vi "Minhee Analysis_new.vi"(4 "Polarity":T2 items=["Inward", "Outward"], 5 "Data type":T1 items=["AXON", "HEKA"], 6 "Sweep length":dbl=51662.0, 7 "Path of File":path=path "C:/Users/KimYG/Desktop/test4.abf") -> ()   [LabVIEW 2017]
uses:
  <vilib>/Analysis/NI_AALBase.lvlib
  <vilib>/addons/_Advanced Signal Processing/NI_AdvSigProcWA.lvlib
  <vilib>/Utility/file.llb/Write Delimited Spreadsheet (DBL).vi
  <vilib>/Utility/miscctls.llb/LVRowAndColumnTypeDef.ctl
  <vilib>/Analysis/3filter.llb/Savitzky-Golay Filter (DBL).vi
  <vilib>/addons/Wavelet Analysis/application.llb/WA Multiscale Peak Detection (Array).vi
  Event Detection cluster.ctl
  <vilib>/Analysis/baseanly.llb/Mean (DBL).vi
  Minhee analysis parameter setting.ctl
  Polarity.ctl
  Data type_new.ctl
panel:
  out "Holding Current":dbl[](graph)
  out "Mean Frequency":string caption="String"
  out "Sweep duration":dbl
  in  "Clipboard":bool
  out "Number of event":i32[][](graph)
  out "Selected event":string caption="String"
  out "Pining point":string caption="String"
  out "Mean IEI":string caption="String"
  out "Mean Amplitude":string caption="String"
  out "Total event":string caption="String"
  in  "Pin here":bool
  in  "Raw trace":bool
  out "Distribution of amplitude 2":T3(graph) caption="Selected"
  out "Distribution of IEI 2":T3(graph) caption="Selected"
  out "Mean IEI":string caption="String"
  out "Mean Amplitude":string caption="String"
  out "CV":dbl[](graph)
  in  "Baseline selection":T4(ring)
  in  "Screening":bool
  out "dv/dt":cluster{"X (time)":dbl[], "dX/dt":dbl[]}[](graph)
  in  "Save":bool
  out "Distribution of amplitude":T3(graph) caption="Total"
  out "Distribution of IEI":T3(graph) caption="Total"
  in  "Event #":i16=4 min=0 max=15 step=1
  out "Event":cluster{dbl[], dbl[]}[](graph)
  in  "Delete":bool
  in  "Do it":bool
  in  "Parameter setting":T5={"Event Detection Parameter"={"Threshold"=-10.0, "width "=20}, "Smoothing Parameter"={"polynomial order"=3, "side points"=20}, "Screening threshold (dV/dt)"=-6000.0, "Screening threshold (amplitude)"=-10.0} {"Screening threshold (amplitude)" format="%#_13g"; "Event Detection Parameter"."Threshold" format="%#_13g"}
  in  "정지":bool
  in  "Sweep #":i32 min=0 max=49 step=1
  out "Detected Event":string[][](table)
  out "Original trace":cluster{"Ramp Pattern":dbl[], "X":dbl[]}[](graph)
  # "Event Table"
  # "Sweep Info."
  # "Data file configuration"
  # "Parameter setting"
  # "Action"
  # "Search parameter"
  # "Home"
  # "Pg Up"
  # "End"
  # "Pg Dn"
  # "Result - Total & Representative (200 events)"
  # "Minhee Analysis for sEPSC/sIPSC"
  # "Whole trace"
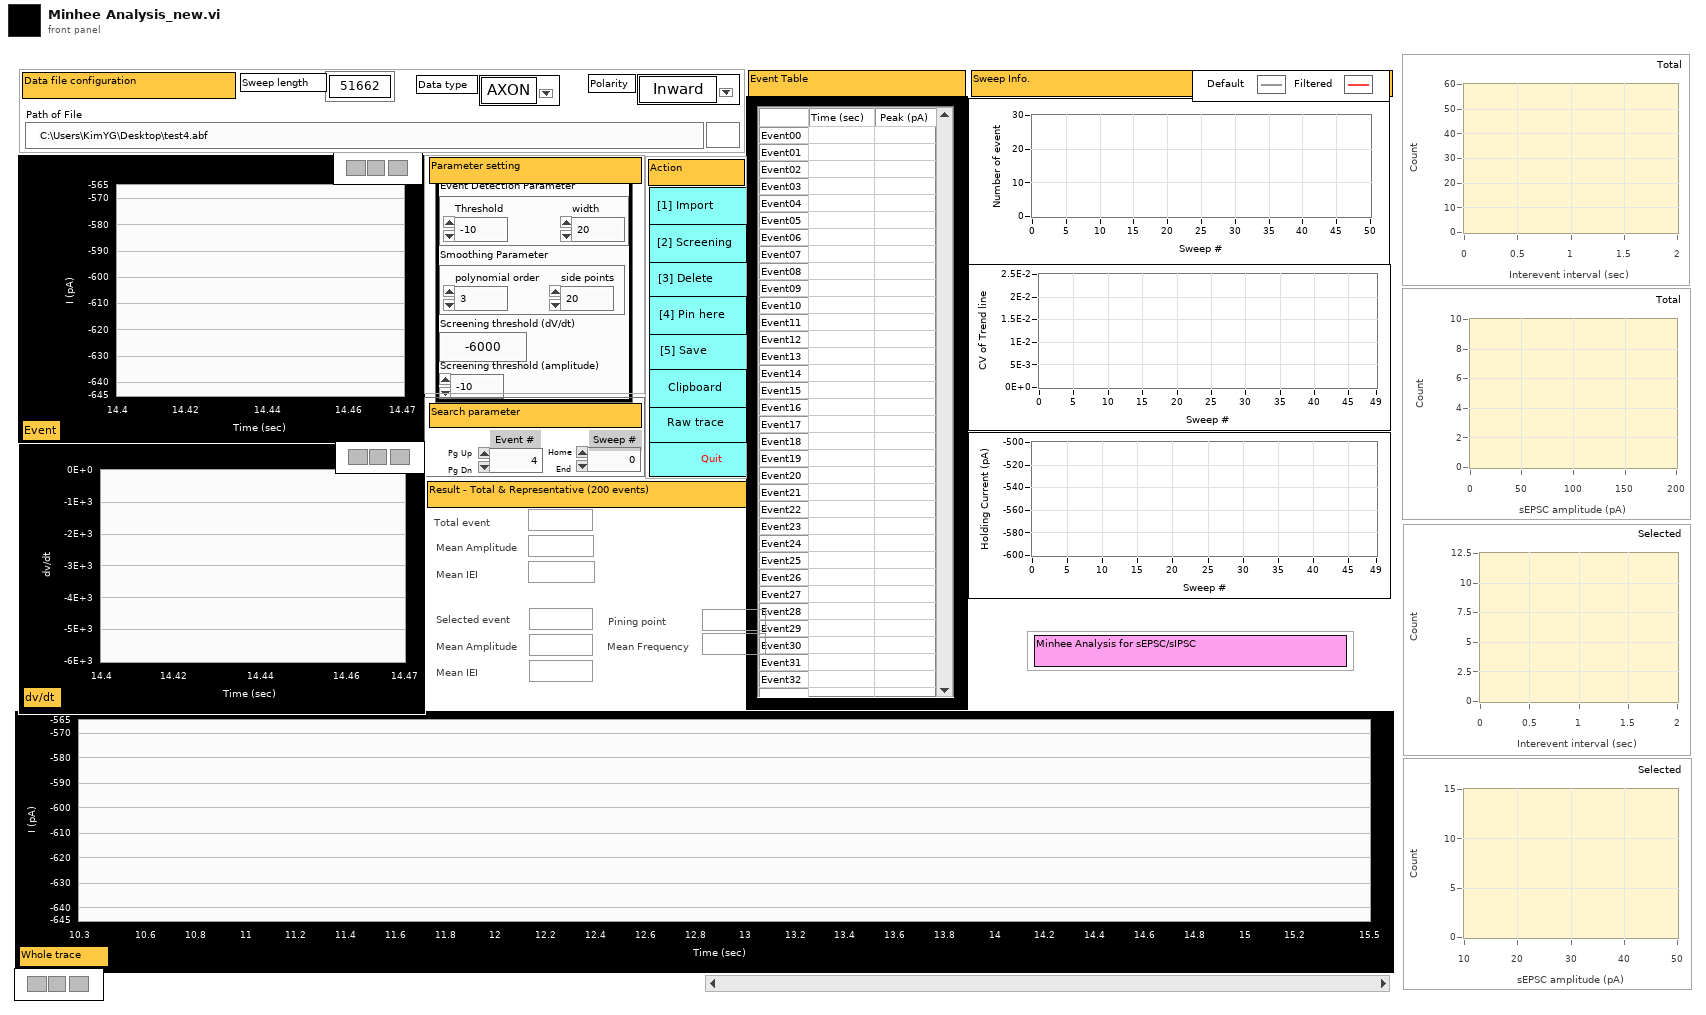
[diagram p1: front panel]
types:
  T1 = typedef "Data type_new.ctl" = u16
  T2 = typedef "Polarity.ctl" = u16
  T3 = cluster{"X Values":dbl[], "Histogram: h(x)":i32[]}
  T4 = enum16{"Adjusted baseline", "Trend line", "Previously used"}
  T5 = typedef "Minhee analysis parameter setting.ctl" = cluster{"Event Detection Parameter":cluster{"Threshold":dbl, "width ":i32}, "Smoothing Parameter":cluster{"polynomial order":i32, "side points":i32}, "Screening threshold (dV/dt)":dbl, "Screening threshold (amplitude)":dbl}
  T6 = typedef "Event Detection cluster.ctl" = cluster{"Event (1D)":cluster{"Event time":dbl[], "Event Peak":dbl[]}, "Trace (1D)":cluster{"Trace time":dbl[], "Trace":dbl[]}, "Trend (1D)":cluster{"Trend time":dbl[], "Trend":dbl[]}, "Baseline (1D)":cluster{"Baseline time":dbl[], "Baseline":dbl[]}}
  T7 = cluster{"Total":cluster{"Distribution of IEI":cluster{"X Values":dbl[], "Histogram: h(x)":i32[]}, "Distribution of amplitude":cluster{"X Values":dbl[], "Histogram: h(x)":i32[]}, "Total":cluster{"EVT #":string, "Amplitude":string, "IEI":string}, "Number of event":i32[]}, "Selected":cluster{"Distribution of IEI ":cluster{"X Values":dbl[], "Histogram: h(x)":i32[]}, "Distribution of amplitude":cluster{"X Values":dbl[], "Histogram: h(x)":i32[]}, "Selected":cluster{"EVT #":string, "Amplitude":string, "IEI":string, "Frequency":string}}}
  T8 = cluster{"X (time)":dbl[], "I (pA)":dbl[], "dX/dt":dbl[]}
  T9 = cluster{"Distribution of IEI ":cluster{"X Values":dbl[], "Histogram: h(x)":i32[]}, "Distribution of amplitude":cluster{"X Values":dbl[], "Histogram: h(x)":i32[]}, "Selected":cluster{"EVT #":string, "Amplitude":string, "IEI":string, "Frequency":string}}
  T10 = cluster{"detrend? (F)":bool, "threshold frequency":dbl}
  T11 = typedef "LVRowAndColumnTypeDef.ctl" = cluster{"Row":i32, "Column":i32}
  T12 = cluster{"File Path":path, "Cell ID":string, "File Name":string, "Total Length":i32, "Trial Length (ms)":dbl, "Sweep Number":dbl, "Sampling rate":dbl}
  T13 = cluster{"polynomial order":i32, "side points":i32}
  T14 = cluster{"Path of File":path, "Sweep length ":dbl, "Data type":T1}
  T15 = cluster{"Histogram Graph":cluster{"X Values":dbl[], "Histogram: h(x)":i32[]}, "Histogram Graph":cluster{"X Values":dbl[], "Histogram: h(x)":i32[]}, cluster{"EVT #":string, "Mean amplitude":string, "Mean IEI":string, "Mean frequency":string}}
  T16 = typedef "Baseline selection.ctl" = enum16{"Default", "Manual"}
  T17 = cluster{"Histogram Graph":cluster{"X Values":dbl[], "Histogram: h(x)":i32[]}, "Histogram Graph":cluster{"X Values":dbl[], "Histogram: h(x)":i32[]}, cluster{string, "standard deviation":string, "standard deviation":string}, i32[]}
  T18 = cluster{"EVT #":string, "Amplitude":string, "IEI":string}
  T19 = cluster{"EVT #":string, "Amplitude":string, "IEI":string, "Frequency":string}
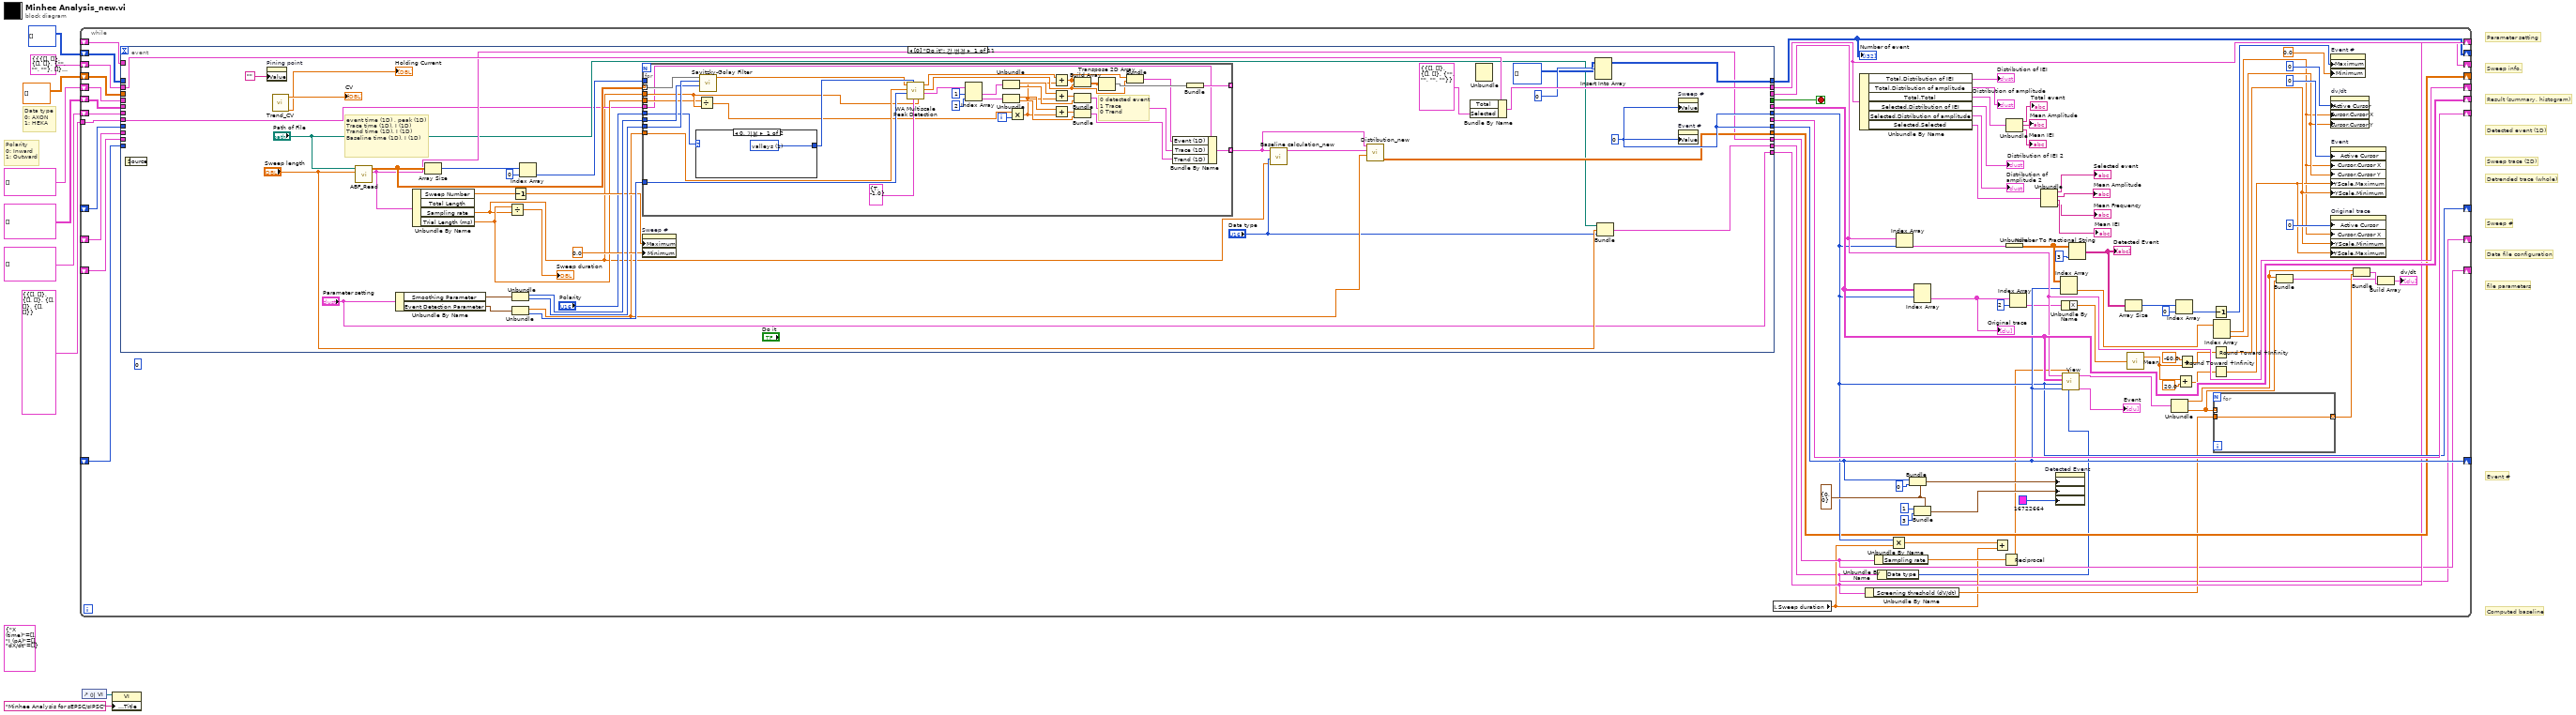
[diagram p0: block diagram]
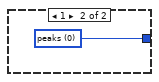
[diagram p2: hidden frame]
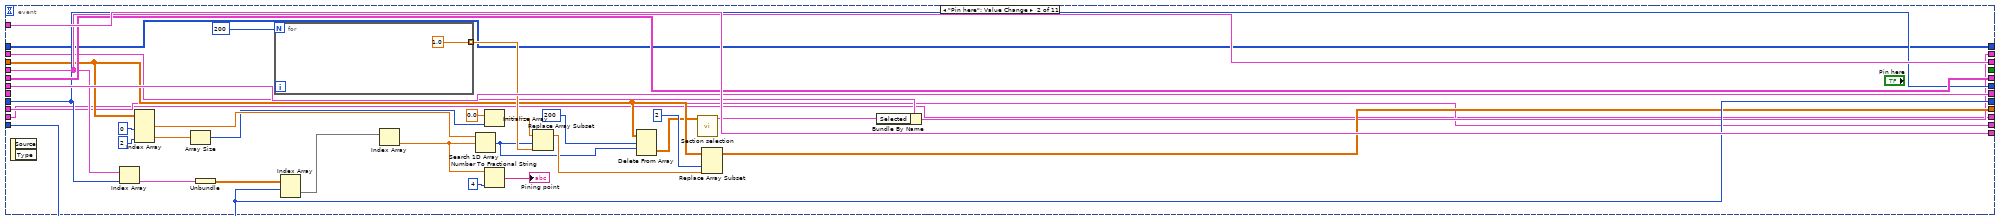
[diagram p3: hidden frame]
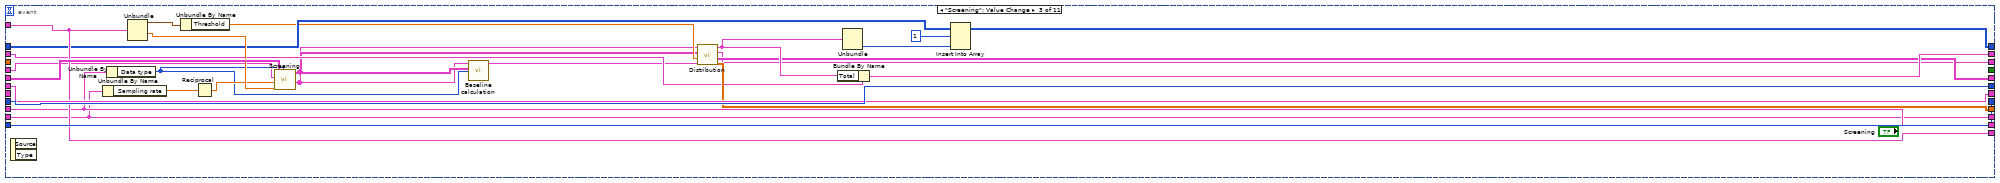
[diagram p4: hidden frame]
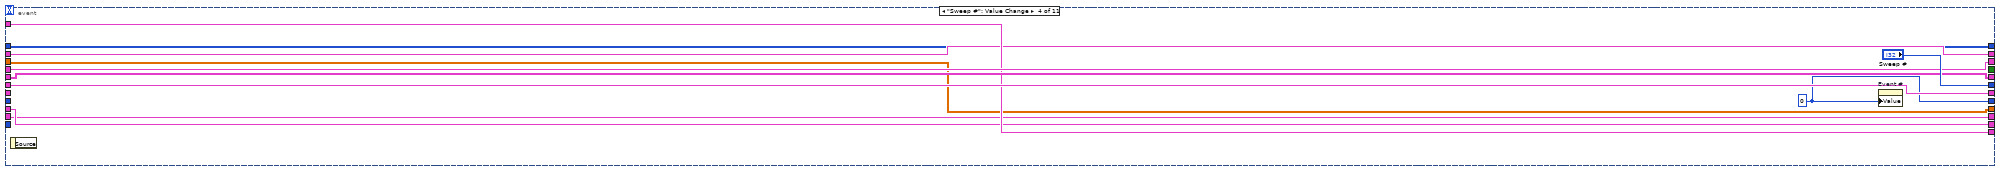
[diagram p5: hidden frame]
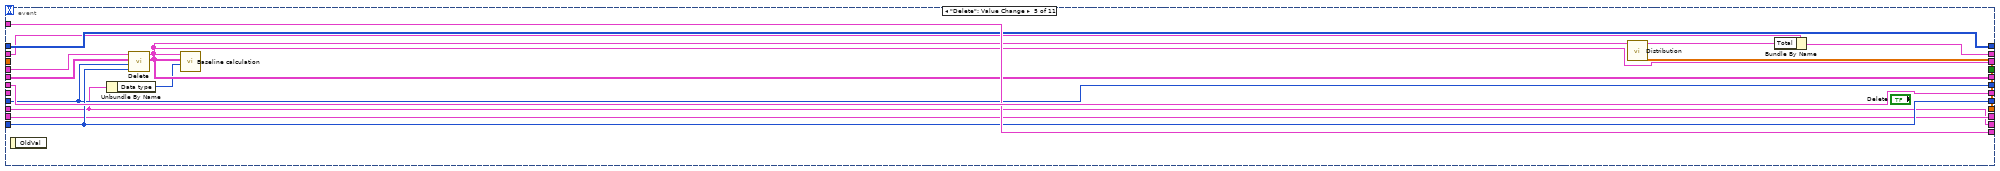
[diagram p6: hidden frame]
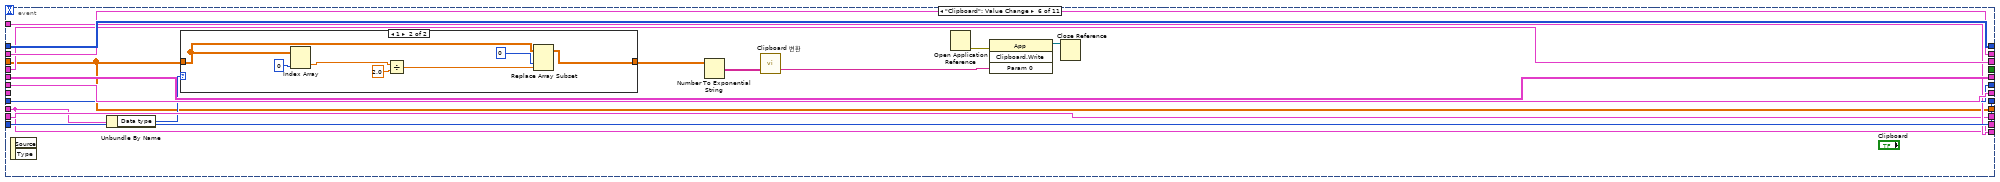
[diagram p7: hidden frame]
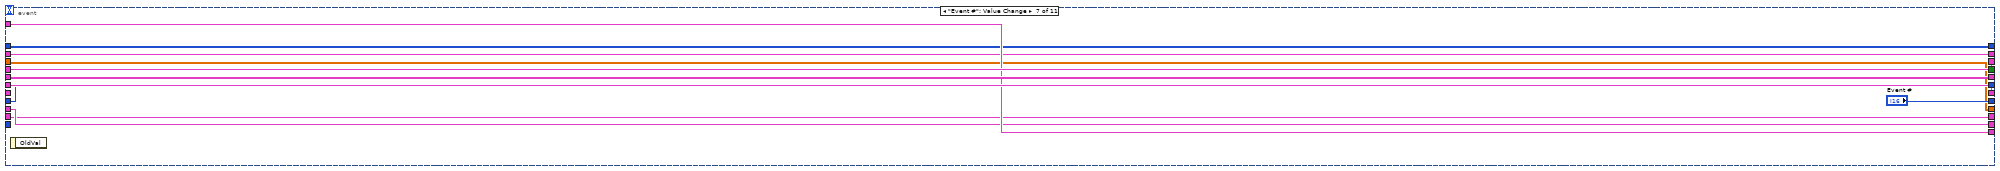
[diagram p9: hidden frame]
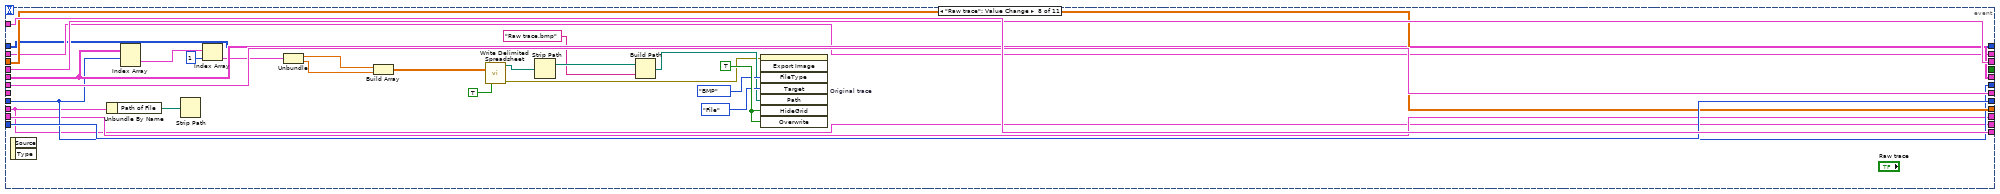
[diagram p10: hidden frame]
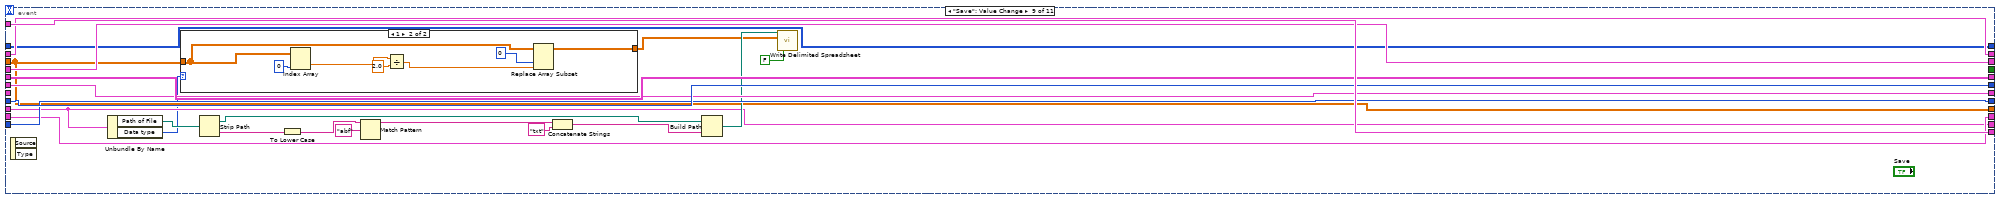
[diagram p11: hidden frame]
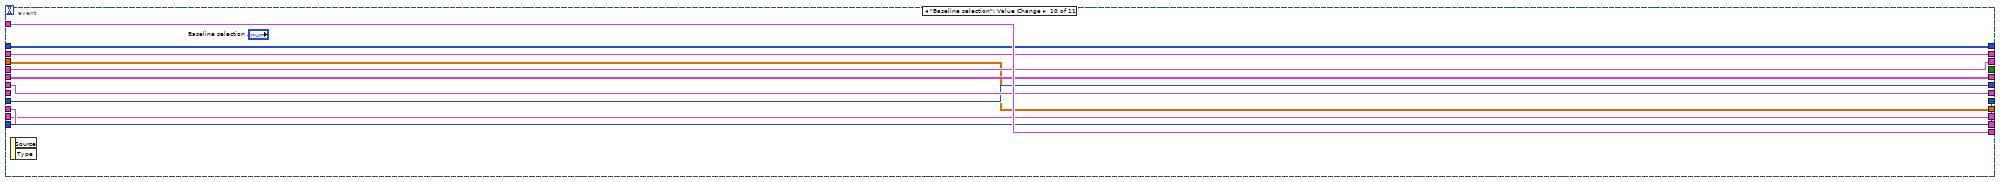
[diagram p13: hidden frame]
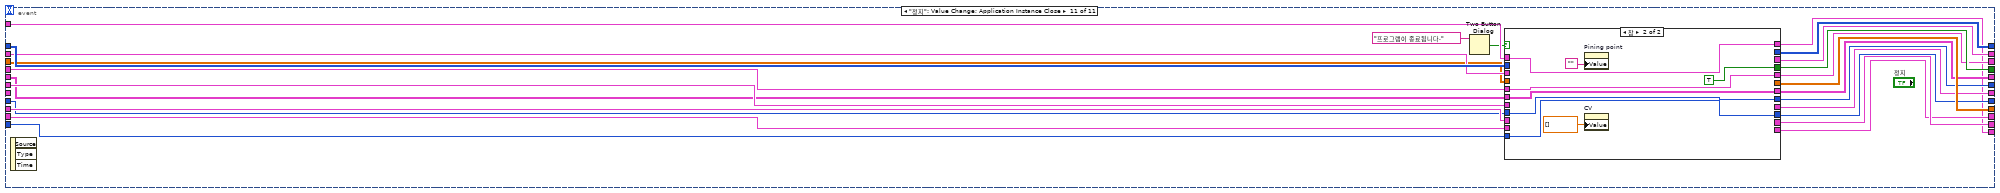
[diagram p14: hidden frame]
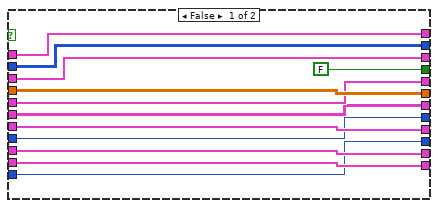
[diagram p15: hidden frame]
diagram:
  (unwired) T8 {"X (time)"=[], "I (pA)"=[], "dX/dt"=[]} ("출력 클러스터")
  # "Polarity \n0: Inward\n1: Outward"
  # "Data type \n0: AXON\n1: HEKA"
  # "file parameters"
  # "Data file configuration"
  # "Parameter setting"
  # "Sweep info."
  # "Result (summary, histogram)"
  # "Computed baseline"
  # "Sweep trace (2D)"
  # "Detrended trace (whole)"
  # "Detected event (1D)"
  # "Event #"
  # "Sweep #"
  n1 = while {
    shift-right: [w82] -> _
    shift-left: cluster{"Ramp Pattern":dbl[], "X":dbl[]}[][] [] ("peak plot") -> [w92]
    shift-right: [w56] -> _
    shift-left: _ -> [w93]
    shift-right: [w78] -> _
    shift-left: cluster{dbl[][]}[] [] -> [w89]
    shift-right: [w87] -> _
    shift-left: cluster{dbl[], dbl[]}[] [] -> [w86]
    shift-right: [w63] -> _
    shift-left: _ -> [w85]
    shift-right: [w46] -> _
    shift-left: _ -> [w83]
    shift-right: [w48] -> _
    shift-left: dbl[][] [] ("Event final") -> [w47]
    shift-right: [w39] -> _
    shift-left: T7 {"Total"={"Distribution of IEI"={"X Values"=[], "Histogram: h(x)"=[]}, "Distribution of amplitude"={"X Values"=[], "Histogram: h(x)"=[]}, "Total"={"EVT #"="", "Amplitude"="", "IEI"=""}, "Number of event"=[]}, "Selected"={"Distribution of IEI "={"X Values"=[], "Histogram: h(x)"=[]}, "Distribution of amplitude"={"X Values"=[], "Histogram: h(x)"=[]}, "Selected"={"EVT #"="", "Amplitude"="", "IEI"="", "Frequency"=""}}} -> [w40]
    shift-right: [w25] -> _
    shift-left: i32[][] [] -> [w26]
    shift-right: [w17] -> _
    shift-left: _ -> [w24]
    shift-right: [w22] -> _
    shift-left: _ -> [w23]
    tunnel: T6 {"Event (1D)"={"Event time"=[], "Event Peak"=[]}, "Trace (1D)"={"Trace time"=[], "Trace"=[]}, "Trend (1D)"={"Trend time"=[], "Trend"=[]}, "Baseline (1D)"={"Baseline time"=[], "Baseline"=[]}} ("Event DEtection") -> [w10]
    stop <- w91 stop-if-true
    (unwired) u32 0 ("활성 커서")
    w58 = T11 {"Row"=0, "Column"=0} ("선택 시작")
    n2 = event shown="[0] \"Do it\": 값 변경" {
      selector: _ -> [_ _ _ _ _ _ _ _ _ _ _]
      dyn-events: _ -> [_ _ _ _ _ _ _ _ _ _ _]
      timeout: _ -> [_ _ _ _ _ _ _ _ _ _ _]
      tunnel: [_ w202 w208 w241 w252 w271 w291 w316 w341 w362 w370] -> w82
      tunnel: [w131 w199 w231 "Sweep #" w253 w269 w292 w315 w343 w358 w366] -> w56
      tunnel: w93 -> [_ w199 w231 _ w253 w269 w292 w315 w343 w358 w378]
      tunnel: w92 -> [_ w202 w228 w241 w256 w271 w291 w316 w341 w362 w371]
      tunnel: [_ _ _ _ _ _ _ _ _ _ w388] -> w91
      tunnel: [_ w200 w206 w240 w249 w272 w290 w319 w340 w361 w372] -> w78
      tunnel: w89 -> [_ w200 w212 w240 w257 w272 w290 w319 w340 w361 w382]
      tunnel: [_ w201 w229 w239 w258 w273 w294 w318 w339 w360 w373] -> w87
      tunnel: w86 -> [_ w201 w229 w239 w258 w273 w294 w318 w339 w360 w383]
      tunnel: [w131 w196 w230 w238 w254 w270 "Event #" w320 w342 w359 w367] -> w63
      tunnel: w85 -> [_ w196 w230 _ w254 w270 _ w320 w342 w359 w379]
      tunnel: w83 -> [_ w203 w226 w237 w255 w268 w289 w321 w344 w363 w377]
      tunnel: ["Parameter setting" w203 w226 w237 w255 w268 w289 w321 w344 w363 w365] -> w46
      tunnel: [w122 w192 w224 w236 w248 w259 w286 w317 w331 w357 w374] -> w48
      tunnel: w47 -> [_ w183 _ w236 _ w259 w286 w317 w331 w357 w384]
      tunnel: w40 -> [w121 w176 w223 w235 w246 w274 w288 w299 w327 w356 w385]
      tunnel: [w120 w174 w222 w235 w245 w274 w288 w299 w327 w356 w375] -> w39
      tunnel: w26 -> [_ w173 w221 w234 w251 w275 w287 w298 w326 w355 w386]
      tunnel: [w119 w173 w220 w234 w251 w275 w287 w298 w326 w355 w376] -> w25
      tunnel: w24 -> [_ w172 w216 w233 w244 w262 w285 w296 w324 w354 w381]
      tunnel: [w107 w172 w216 w233 w244 w262 w285 w296 w324 w354 w369] -> w17
      tunnel: [w116 w171 w215 w232 w250 w263 w284 w297 w325 w353 w368] -> w22
      tunnel: w23 -> [_ w171 w215 w232 w250 w263 w284 w297 w325 w353 w380]
      tunnel: w10 -> [w98 _ _ _ _ _ _ _ _ _ _]
      event "Do it": Value Change {
        w131 = i16 0 ("Event #")
        # "event time (1D) , peak (1D)\nTrace time (1D), I (1D)\nTrand time (1D), I (1D)\nBaseline time (1D), I (1D)"
        n3 = event-data() -> ()  [unwired: 1 in, 1 out]
        n4 = property on="Pining point" class="Str"("Value"="") -> ()  [unwired: 2 in, 2 out]
        n5 = call "Trend_CV.vi"() -> ("Holding Current (pA)"=→"Holding Current":dbl[], "CV"=→"CV":dbl[])  [unwired: 6 in]
        n6 = call "ABF_Read.vi"("Trial Length (ms)"="Sweep length", "Path of ABF file"="Path of File") -> ("File Paramters"=w116:T12, "Whole Trace"=w117:dbl[][])  [unwired: 2 in, 2 out]
        n7 = Unbundle By Name("Parameter setting") -> ("Smoothing Parameter"=w128:T13, "Event Detection Parameter"=w130:cluster{"Threshold":dbl, "width ":i32})
        n8 = Unbundle By Name(w116) -> ("Sweep Number"=w114:dbl, "Sampling rate"=w97:dbl, "Trial Length (ms)"=w112:dbl)  [unwired: 1 out]
        n9 = Array Size(array=w117) -> (size(s)=w125:i32[])
        n10 = Divide(x=w112, y=w97) -> (x/y=→"Sweep duration":dbl)
        n11 = Unbundle(w128) -> ("polynomial order"=w127:i32, "side points"=w126:i32)
        n12 = Unbundle(w130) -> ("Threshold"=w102:dbl, "width"=w129:i32)
        n13 = Decrement(x=w114) -> (x-1=w115:dbl)
        n14 = Index Array(array=w125, index=0 ("인덱스")) -> (element=w123:i32)
        n15 = for {
          tunnel: w117 -> [w167] mode=indexing
          tunnel: w97 -> [w160]
          tunnel: w126 -> [w164]
          tunnel: w127 -> [w163]
          tunnel: w102 -> [w162]
          tunnel: w129 -> [w161]
          tunnel: w112 -> [w151]
          tunnel: [w154] -> _ mode=indexing
          tunnel: w123 -> [_]
          tunnel: "Polarity" -> [w137]
          tunnel: w98 -> [w136]
          tunnel: [w132] -> w95 mode=indexing
          i -> [w138]
          # "0 detected event\n1 Trace\n0 Trend"
          n16 = case shown="0, 기본" w137 {
            tunnel: [w168 w169] -> w166
            frame 0, Default {
              w168 = u16 1 items=["peaks", "valleys"] ("peaks/valleys")
            }
            frame 1 {
              w169 = u16 0 items=["peaks", "valleys"] ("peaks/valleys")
            }
          }
          n17 = Divide(x=w151, y=w160) -> (x/y=w159:dbl)
          n18 = call-poly <vilib>:"Savitzky-Golay Filter.vi"("polynomial order"=w163, "side points"=w164, "X"=w167) -> ("Filtered X"=w158:dbl[])  [unwired: 7 in, 1 out]
          n19 = call-poly <vilib>:"WA Multiscale Peak Detection.vi"("sampling rate"=w160, "detrend settings"=T10 {"detrend? (F)"=TRUE, "threshold frequency"=-1.0}, "peaks/valleys"=w166, "width"=w161, "threshold"=w162, "signal"=w158) -> ("peak plot"=w150:cluster{"Ramp Pattern":dbl[], "X":dbl[]}[], "amplitude"=w152:dbl[], "location"=w157:dbl[])  [unwired: 1 in, 2 out]
          n20 = Index Array(array=w150, index #1=1 ("인덱스"), index #2=2 ("인덱스")) -> (element #1=w148:cluster{"Ramp Pattern":dbl[], "X":dbl[]}, element #2=w143:cluster{"Ramp Pattern":dbl[], "X":dbl[]})
          n21 = Unbundle(w148) -> ("Ramp Pattern"=w147:dbl[], "X"=w145:dbl[])
          n22 = Unbundle(w143) -> ("Ramp Pattern"=w142:dbl[], "X"=w140:dbl[])
          n23 = Multiply(x=w159, y=w138) -> (x*y=w139:dbl)
          n24 = Add(x=w157, y=w139) -> (x+y=w153:dbl[])
          n25 = Add(x=w147, y=w139) -> (x+y=w146:dbl[])
          n26 = Add(x=w142, y=w139) -> (x+y=w141:dbl[])
          n27 = Build Array(w153, w152) -> (w156:dbl[][])
          n28 = Bundle(w146, "X"=w145) -> (w134:cluster{dbl[], "X":dbl[]})  [unwired: 1 in]
          n29 = Bundle(w141, "X"=w140) -> (w133:cluster{dbl[], "X":dbl[]})  [unwired: 1 in]
          n30 = Transpose 2D Array(2D array=w156) -> (transposed array=w155:dbl[][])
          n31 = Bundle(w153, "amplitude"=w152) -> (w135:cluster{dbl[], "amplitude":dbl[]})  [unwired: 1 in]
          n32 = Bundle By Name(cluster=w136, "Event (1D)"=w135, "Trace (1D)"=w134, "Trend (1D)"=w133) -> (w132:T6)
          n33 = Bundle(w155) -> (w154:cluster{dbl[][]})  [unwired: 1 in]
        }
        n34 = property on="Sweep #" class="DigNum (엄격한)"("Maximum"=w115, "Minimum"=0.0 ("데이터 입력 제한:최소")) -> ()  [unwired: 2 in, 2 out]
        n35 = call "Baseline calculation_new.vi"("Sampling rate"=w97, "Data type"="Data type", "Event Detection (1D)"=w95) -> ("Baseline info"=w96:cluster{dbl[][]}[])  [unwired: 4 in]
        n36 = call "Distribution_new.vi"("Threshold"=w102, "Baseline info 2"=w96, "Event Detection (1D)"=w95) -> ("Event final"=w122:dbl[][])  [unwired: 2 in, 2 out]
        n37 = Bundle By Name(cluster=w121, "Selected"=T9 {"Distribution of IEI "={"X Values"=[], "Histogram: h(x)"=[]}, "Distribution of amplitude"={"X Values"=[], "Histogram: h(x)"=[]}, "Selected"={"EVT #"="", "Amplitude"="", "IEI"="", "Frequency"=""}}) -> (w120:T7)  [unwired: 1 in]
        n38 = Unbundle() -> ()  [unwired: 1 in, 4 out]
        n39 = Insert Into Array(array=i32[][] [], index (row)=0) -> (w119:i32[][])  [unwired: 2 in]
        n40 = Bundle("Path of File"="Path of File", "Sweep length"="Sweep length", "Data type"="Data type") -> (w107:T14)  [unwired: 1 in]
        n41 = property on="Sweep #" class="DigNum (엄격한)"("Value"=w131) -> ()  [unwired: 2 in, 2 out]
        n42 = property on="Event #" class="DigNum (엄격한)"("Value"=w131) -> ()  [unwired: 2 in, 2 out]
      }
      event "Pin here": Value Change {
        n43 = event-data() -> ()  [unwired: 1 in, 2 out]
        n44 = Index Array(array=w200, index=w199) -> (element=w198:cluster{dbl[][]})
        n45 = Index Array(array=w183, index (col) #1=0 ("비활성화된 인덱스 (열)"), index (col) #2=2 ("인덱스 (열)")) -> (element #1=w193:dbl[], element #2=w187:dbl[])  [unwired: 2 in]
        n46 = Array Size(array=w187) -> (size(s)=w186:i32)
        n47 = Unbundle(w198) -> (w197:dbl[][])
        n48 = for {
          N: 200 -> [_]
          tunnel: [1.0 ("x")] -> w190 mode=indexing
        }
        n49 = Index Array(array=w197, index (row)=w196) -> (element=w195:dbl[])  [unwired: 1 in]
        n50 = Index Array(array=w195) -> (element=w179:dbl)  [unwired: 1 in]
        n51 = Search 1D Array(1D array=w193, element=w179) -> (index of element=w181:i32)  [unwired: 1 in]
        n52 = Initialize Array(0.0 ("원소"), w186) -> (w184:dbl[])
        n53 = Number To Fractional String(number=w179, precision (6)=i16 4 ("정밀도(6)")) -> (F-format string=→"Pining point":string)  [unwired: 2 in]
        n54 = Replace Array Subset(array=w184, new element=w190, index=w181) -> (w188:dbl[])
        n55 = Delete From Array(array=w183, length=200 ("길이"), index (row)=w181) -> (deleted portion=w180:dbl[][])  [unwired: 1 in, 1 out]
        n56 = call "Section selection.vi"("Event final"=w180) -> ("Distribution (output)"=w175:T15)  [unwired: 6 in]
        n57 = Replace Array Subset(array=w183, new element=w188, index (col)=2 ("비활성화된 인덱스 (열)")) -> (w192:dbl[][])  [unwired: 1 in]
        n58 = Bundle By Name(cluster=w176, "Selected"=w175) -> (w174:T7)
      }
      event "Screening": Value Change {
        n59 = event-data() -> ()  [unwired: 1 in, 2 out]
        n60 = Unbundle By Name(w215) -> ("Sampling rate"=w214:dbl)
        n61 = Unbundle By Name(w216) -> ("Data type"=w213:T1)
        n62 = Unbundle(w226) -> ("Event Detection Parameter"=w211:cluster{"Threshold":dbl, "width ":i32}, "Screening threshold (dV/dt)"=w227:dbl)  [unwired: 2 out]
        n63 = Unbundle By Name(w211) -> ("Threshold"=w210:dbl)
        n64 = Reciprocal(x=w214) -> (1/x=w225:dbl)
        n65 = call "Screening.vi"("Data type"=w213, "Screen threshold (dV/dt)"=w227, "dt"=w225, "Detected Event (1D) In"=w212, "Sweep trace (2D) In"=w228) -> ("Detected Event (1D) Out"=w207:cluster{dbl[][]}[], "Sweep trace (2D) Out"=w209:cluster{"Ramp Pattern":dbl[], "X":dbl[]}[][])  [unwired: 2 in]
        n66 = call "Baseline calculation.vi"("Data type"=w213, "Sweep trace (2D) In"=w209, "Detected Event (1D) In"=w207) -> ("Baseline info"=w205:cluster{T16[], dbl[]}[])  [unwired: 3 in, 1 out]
        n67 = call "Distribution.vi"("Detected Event (1D)"=w207, "Sweep trace (2D) In"=w209, "Threshold"=w210, "Baseline info new"=w205) -> ("Distribution (output)"=w218:T17, "Detected Event (1D) OUT"=w206:cluster{dbl[][]}[], "Sweep trace (2D) Out"=w208:cluster{"Ramp Pattern":dbl[], "X":dbl[]}[][], "Event final"=w224:dbl[][])  [unwired: 1 out]
        n68 = Bundle By Name(cluster=w223, "Total"=w218) -> (w222:T7)
        n69 = Unbundle(w218) -> (w217:i32[])  [unwired: 3 out]
        n70 = Insert Into Array(array=w221, index (row)=1, new element=w217) -> (w220:i32[][])  [unwired: 1 in]
      }
      event "Sweep #": Value Change {
        w238 = i16 0 ("Event #")
        n71 = event-data() -> ()  [unwired: 1 in, 1 out]
        n72 = property on="Event #" class="DigNum (엄격한)"("Value"=w238) -> ()  [unwired: 2 in, 2 out]
      }
      event "Delete": Value Change {
        n73 = event-data() -> ()  [unwired: 1 in, 1 out]
        n74 = Unbundle By Name(w244) -> ("Data type"=w243:T1)
        n75 = call "Delete.vi"("Event #"=w254, "Sweep #"=w253, "Sweep trace (2D) In"=w256, "Detected Event (1D) In"=w257) -> ("Sweep trace (2D) Out"=w252:cluster{"Ramp Pattern":dbl[], "X":dbl[]}[][], "Detected Event (1D) Out"=w249:cluster{dbl[][]}[])  [unwired: 2 in]
        n76 = call "Baseline calculation.vi"("Data type"=w243, "Sweep trace (2D) In"=w252, "Detected Event (1D) In"=w249) -> ()  [unwired: 3 in, 2 out]
        n77 = call "Distribution.vi"("Detected Event (1D)"=w249) -> ("Distribution (output)"=w247:T17, "Event final"=w248:dbl[][])  [unwired: 3 in, 3 out]
        n78 = Bundle By Name(cluster=w246, "Total"=w247) -> (w245:T7)
      }
      event "Clipboard": Value Change {
        n79 = event-data() -> ()  [unwired: 1 in, 2 out]
        n80 = Unbundle By Name(w262) -> ("Data type"=w261:T1)
        n81 = case shown="1" w261 {
          tunnel: w259 -> [w276 w283]
          tunnel: [w276 w282] -> w260
          frame 0, Default {
          }
          frame 1 {
            n82 = Index Array(array=w283, index (col)=0 ("비활성화된 인덱스 (열)")) -> (element=w280:dbl[])  [unwired: 1 in]
            n83 = Divide(x=w280, y=2.0 ("x")) -> (x/y=w278:dbl[])
            n84 = Replace Array Subset(array=w283, new element=w278, index (col)=0 ("비활성화된 인덱스 (열)")) -> (w282:dbl[][])  [unwired: 1 in]
          }
        }
        n85 = Number To Exponential String(number=w260) -> (E-format string=w264:string[][])  [unwired: 3 in]
        n86 = call "Clipboard 변환.vi"("Input (structured)"=w264) -> ("Output (flattened)"=w265:string)  [unwired: 1 in, 1 out]
        n87 = Open Application Reference() -> (0:w267:errorcluster)  [unwired: 4 in, 1 out]
        n88 = invoke class="App" method="Clipboard.Write"(error in=w267, "Param 0"=w265) -> (reference out=w266:refnum<vi>)  [unwired: 2 in, 3 out]
        n89 = Close Reference(reference=w266) -> ()  [unwired: 1 in, 1 out]
      }
      event "Event #": Value Change {
        n90 = event-data() -> ()  [unwired: 1 in, 1 out]
      }
      event "Raw trace": Value Change {
        w307 = TRUE ("눈금 숨기기")
        n91 = event-data() -> ()  [unwired: 1 in, 2 out]
        n92 = Unbundle By Name(w296) -> ("Path of File"=w295:path)
        n93 = Index Array(array=w316, index (row)=w315) -> (element=w314:cluster{"Ramp Pattern":dbl[], "X":dbl[]}[])  [unwired: 1 in]
        n94 = Strip Path(path=w295) -> ()  [unwired: 2 out]
        n95 = Index Array(array=w314, index=1 ("인덱스")) -> (element=w312:cluster{"Ramp Pattern":dbl[], "X":dbl[]})
        n96 = Unbundle(w312) -> ("Ramp Pattern"=w311:dbl[], "X"=w310:dbl[])
        n97 = Build Array(w311, w310) -> (w309:dbl[][])
        n98 = call-poly <vilib>:"Write Delimited Spreadsheet.vi"("2D data"=w309, "transpose? (no:F)"=TRUE ("transpose? (F)")) -> ("new file path (Not A Path if cancelled)"=w304:path, "error out"=w300:errorcluster)  [unwired: 12 in]
        n99 = Strip Path(path=w304) -> (stripped path=w303:path)  [unwired: 1 out]
        n100 = Build Path(base path=w303, name or relative path="Raw trace.bmp" ("이름 또는 상대 경로")) -> (appended path=w301:path)
        n101 = invoke on="Original trace" class="XYGraph (엄격한)" method="Export Image"(error in=w300, "FileType"=enum32{"BMP", "EPS", "EMF", "PICT"}."BMP" ("파일 타입"), "Target"=enum32{"File", "Clipboard"}."File" ("타겟"), "Path"=w301, "HideGrid"=w307, "Overwrite"=w307) -> ()  [unwired: 2 in, 8 out]
      }
      event "Save": Value Change {
        n102 = event-data() -> ()  [unwired: 1 in, 2 out]
        n103 = Unbundle By Name(w324) -> ("Path of File"=w323:path, "Data type"=w322:T1)
        n104 = case shown="1" w322 {
          tunnel: w331 -> [w345 w352]
          tunnel: [w345 w351] -> w330
          frame 0, Default {
          }
          frame 1 {
            n105 = Index Array(array=w352, index (col)=0 ("비활성화된 인덱스 (열)")) -> (element=w349:dbl[])  [unwired: 1 in]
            n106 = Divide(x=w349, y=2.0 ("x")) -> (x/y=w347:dbl[])
            n107 = Replace Array Subset(array=w352, new element=w347, index (col)=0 ("비활성화된 인덱스 (열)")) -> (w351:dbl[][])  [unwired: 1 in]
          }
        }
        n108 = Strip Path(path=w323) -> (stripped path=w333:path, name=w329:string)
        n109 = To Lower Case(string=w329) -> (all lower case string=w328:string)
        n110 = Match Pattern(string=w328, regular expression="abf" ("정규식")) -> (before substring=w336:string)  [unwired: 1 in, 3 out]
        n111 = Concatenate Strings(w336, "txt" ("문자열")) -> (w334:string)
        n112 = Build Path(base path=w333, name or relative path=w334) -> (appended path=w332:path)
        n113 = call-poly <vilib>:"Write Delimited Spreadsheet.vi"("file path (dialog if empty)"=w332, "2D data"=w330, "transpose? (no:F)"=FALSE ("transpose? (F)")) -> ()  [unwired: 11 in, 2 out]
      }
      event "Baseline selection": Value Change {
        n114 = event-data() -> ()  [unwired: 1 in, 2 out]
      }
      event "정지": Value Change; Application Instance Close {
        n115 = event-data() -> ()  [unwired: 1 in, 3 out]
        n116 = Two Button Dialog(message="프로그램이 종료됩니다." ("메시지")) -> (T button?=w364:bool)  [unwired: 2 in]
        n117 = case shown="참" w364 {
          tunnel: [FALSE TRUE] -> w388
          tunnel: w386 -> [w400 _]
          tunnel: w385 -> [w399 _]
          tunnel: w384 -> [w398 _]
          tunnel: w383 -> [w397 _]
          tunnel: w382 -> [w396 w401]
          tunnel: w381 -> [w394 _]
          tunnel: w380 -> [w393 _]
          tunnel: w379 -> [w392 w405]
          tunnel: w378 -> [w391 w404]
          tunnel: w377 -> [w390 w403]
          tunnel: [w400 _] -> w376
          tunnel: [w399 _] -> w375
          tunnel: [w398 _] -> w374
          tunnel: [w397 _] -> w373
          tunnel: [w396 w401] -> w372
          tunnel: w371 -> [w395 w406]
          tunnel: [w395 w406] -> w370
          tunnel: [w394 _] -> w369
          tunnel: [w393 _] -> w368
          tunnel: [w392 w405] -> w367
          tunnel: [w391 w404] -> w366
          tunnel: [w390 w403] -> w365
          frame False {
          }
          frame True {
            n118 = property on="Pining point" class="Str"("Value"="") -> ()  [unwired: 2 in, 2 out]
            n119 = property on="CV" class="WFGraph (엄격한)"("Value"=dbl[] [] ("CV")) -> ()  [unwired: 2 in, 2 out]
          }
        }
      }
    }
    "Number of event" <- w25
    n120 = local read "Sweep duration"() -> (w19:dbl)
    n121 = Unbundle By Name(w39) -> ("Total.Distribution of IEI"=→"Distribution of IEI":T3, "Total.Distribution of amplitude"=→"Distribution of amplitude":T3, "Total.Total"=w36:T18, "Selected.Distribution of IEI"=→"Distribution of IEI 2":T3, "Selected.Distribution of amplitude"=→"Distribution of amplitude 2":T3, "Selected.Selected"=w30:T19)
    n122 = Unbundle By Name(w46) -> ("Screening threshold (dV/dt)"=w45:dbl)
    n123 = Unbundle By Name(w22) -> ("Sampling rate"=w21:dbl)
    n124 = Unbundle By Name(w17) -> ("Data type"=w16:T1)
    n125 = Multiply(x=w56, y=w19) -> (x*y=w90:dbl)
    n126 = Index Array(array=w78, index=w56) -> (element=w88:cluster{dbl[][]})
    n127 = Bundle(cluster=w58, "Row"=w63, "Column"=u32 0 ("활성 커서")) -> (w62:T11)
    n128 = Index Array(array=w82, index (row)=w56) -> (element=w54:cluster{"Ramp Pattern":dbl[], "X":dbl[]}[])  [unwired: 1 in]
    "Original trace" <- w54
    n129 = Bundle(cluster=w58, "Row"=u32 1 ("활성 커서"), "Column"=u32 3 ("활성 커서")) -> (w61:T11)
    n130 = Add(x=w90, y=w19) -> ()  [unwired: 1 out]
    n131 = Reciprocal(x=w21) -> (1/x=w20:dbl)
    n132 = Unbundle(w36) -> ("EVT #"=→"Total event":string, "Amplitude"=→"Mean Amplitude":string, "IEI"=→"Mean IEI":string)
    n133 = Unbundle(w88) -> (w66:dbl[][])
    n134 = Index Array(array=w54, index=2 ("인덱스")) -> (element=w52:cluster{"Ramp Pattern":dbl[], "X":dbl[]})
    n135 = Unbundle(w30) -> ("EVT #"=→"Selected event":string, "Amplitude"=→"Mean Amplitude":string, "IEI"=→"Mean IEI":string, "Frequency"=→"Mean Frequency":string)
    n136 = property on="Detected Event" class="Tbl (엄격한)"("Selection Start"=w62, "Selection Size"=w61, "Selection Color"=u32 16722664) -> ()  [unwired: 2 in, 2 out]
    n137 = Index Array(array=w66, index (row)=w63) -> (element=w65:dbl[])  [unwired: 1 in]
    n138 = Unbundle By Name(w52) -> ("X"=w51:dbl[])
    n139 = call "View.vi"("Data type"=w16, "dt"=w20, "Event #"=w63, "Sweep #"=w56, "Sweep trace (2D) In"=w82, "Detected Event (1D) In"=w78) -> ("event"=→"Event":cluster{dbl[], dbl[]}[], "출력 클러스터"=w81:T8)  [unwired: 1 in, 1 out]
    n140 = Number To Fractional String(number=w66, precision (6)=i16 3 ("폭(-)")) -> (F-format string=w67:string[][])  [unwired: 2 in]
    "Detected Event" <- w67
    n141 = Array Size(array=w67) -> (size(s)=w80:i32[])
    n142 = call-poly <vilib>:"Mean.vi"("X"=w51) -> ("mean"=w41:dbl)  [unwired: 1 out]
    n143 = Unbundle(w81) -> ("X (time)"=w76:dbl[], "dX/dt"=w77:dbl[])  [unwired: 1 out]
    n144 = Index Array(array=w80, index=0 ("인덱스 (행)")) -> (element=w71:i32)
    n145 = Add(x=w41, y=20.0 ("x")) -> (x+y=w42:dbl)
    n146 = Add(x=-60.0, y=w41) -> (x+y=w43:dbl)
    n147 = Decrement(x=w71) -> (x-1=w70:i32)
    n148 = Round Toward +Infinity(x=w43) -> (ceil(x): smallest int >= x=w15:dbl)
    n149 = Round Toward +Infinity(x=w42) -> (ceil(x): smallest int >= x=w14:dbl)
    n150 = Index Array(array=w65) -> (element #1=w11:dbl, element #2=w12:dbl)  [unwired: 2 in]
    n151 = for {
      tunnel: w77 -> [_] mode=indexing
      tunnel: [w94] -> w75 mode=indexing
      tunnel: w45 -> [w94]
    }
    n152 = Bundle("X (time)"=w76, "dX/dt"=w77) -> (w73:cluster{"X (time)":dbl[], "dX/dt":dbl[]})  [unwired: 1 in]
    n153 = property on="Event #" class="DigNum (엄격한)"("Maximum"=w70, "Minimum"=0.0 ("데이터 입력 제한:최소")) -> ()  [unwired: 2 in, 2 out]
    n154 = property on="dv/dt" class="XYGraph (엄격한)"("Active Cursor"=u32 0 ("활성 커서"), "Cursor.Cursor X"=w11, "Cursor.Cursor Y"=w12) -> ()  [unwired: 2 in, 2 out]
    n155 = property on="Event" class="XYGraph (엄격한)"("Active Cursor"=u32 0 ("활성 커서"), "Cursor.Cursor X"=w11, "Cursor.Cursor Y"=w12, "YScale.Maximum"=w14, "YScale.Minimum"=w15) -> ()  [unwired: 2 in, 2 out]
    n156 = property on="Original trace" class="XYGraph (엄격한)"("Active Cursor"=u32 0 ("활성 커서"), "Cursor.Cursor X"=w11, "YScale.Minimum"=w15, "YScale.Maximum"=w14) -> ()  [unwired: 2 in, 2 out]
    n157 = Bundle("X (time)"=w76, w75) -> (w74:cluster{"X (time)":dbl[], dbl[]})  [unwired: 1 in]
    n158 = Build Array(w73, w74) -> (→"dv/dt":cluster{"X (time)":dbl[], "dX/dt":dbl[]}[])
  }
  n159 = control-ref of="이 VI"() -> (w5:refnum<vi>)
  n160 = property class="VI"(reference=w5, "Front Panel.Title"="Minhee Analysis for sEPSC/sIPSC" ("프런트패널 윈도우:제목")) -> ()  [unwired: 1 in, 2 out]
